vi "Dresden R2R Sputter 03.02.2018 IY24.vi"() -> ()   [LabVIEW 2009] (continued)
              }
            }
          }
          frame #3 {
            # "ROUTINE CHECK"
            n22291 = local read "Semi"() -> (w23224:bool)
            n22292 = case shown="False" w23224 {
              frame #0 {
                n22293 = stacked-sequence {
                  frame #0 {
                    n22294 = local read "Semi"() -> (w23225:bool)
                    n22295 = case shown="False" w23225 {
                      frame #0 {
                        w23226 = TRUE ("Visible")
                        n22296 = local write "system_status"("Start up was completed." ("system_status")) -> ()
                        n22297 = property on="final_mes_tab" class="TabCtl (strict)"("Visible"=w23226) -> ()  [unwired: 2 in, 2 out]
                        n22298 = local write "Cnt_Do_Buzzer"(w23226) -> ()
                        n22299 = Wait (ms)(milliseconds to wait=u32 3000 ("millisecond multiple")) -> ()  [unwired: 1 out]
                      }
                      frame #1 {
                      }
                    }
                  }
                  frame #1 {
                    n22300 = local read "Semi"() -> (w23229:bool)
                    n22301 = case shown="False" w23229 {
                      frame #0 {
                        w23230 = FALSE ("Visible")
                        n22302 = local write "system_status"("" ("system_status")) -> ()
                        n22303 = Wait (ms)(milliseconds to wait=u32 3000 ("millisecond multiple")) -> ()  [unwired: 1 out]
                        n22304 = local write "Start_up_ch4"(w23230) -> ()
                        n22305 = local write "Cnt_Do_Buzzer"(w23230) -> ()
                        n22306 = property on="final_mes_tab" class="TabCtl (strict)"("Visible"=w23230) -> ()  [unwired: 2 in, 2 out]
                      }
                      frame #1 {
                      }
                    }
                  }
                  frame #2 {
                    n22307 = local read "Semi"() -> (w23233:bool)
                    n22308 = case shown="False" w23233 {
                      frame #0 {
                        n22309 = stacked-sequence {
                          frame #0 {
                            n22310 = local write "Pps_code_entry"("PF331=" ("system_status")) -> ()
                          }
                          frame #1 {
                            n22311 = Wait (ms)(milliseconds to wait=u32 500) -> ()  [unwired: 1 out]
                          }
                          frame #2 {
                            n22312 = local write "Ppsok"(TRUE ("Ppsok")) -> ()
                          }
                          frame #3 {
                            n22313 = Wait (ms)(milliseconds to wait=u32 1000) -> ()  [unwired: 1 out]
                          }
                        }
                      }
                      frame #1 {
                      }
                    }
                  }
                  frame #3 {
                    n22314 = local read "Semi"() -> (w23238:bool)
                    n22315 = case shown="False" w23238 {
                      frame #0 {
                        n22316 = stacked-sequence {
                          frame #0 {
                            n22317 = local write "Pps_code_entry"("PF227=" ("system_status")) -> ()
                          }
                          frame #1 {
                            n22318 = Wait (ms)(milliseconds to wait=u32 500) -> ()  [unwired: 1 out]
                          }
                          frame #2 {
                            n22319 = local write "Ppsok"(TRUE ("Ppsok")) -> ()
                          }
                          frame #3 {
                            n22320 = Wait (ms)(milliseconds to wait=u32 1000) -> ()  [unwired: 1 out]
                          }
                        }
                      }
                      frame #1 {
                      }
                    }
                  }
                  frame #4 {
                    n22321 = local read "Semi"() -> (w23243:bool)
                    n22322 = case shown="False" w23243 {
                      frame #0 {
                        n22323 = stacked-sequence {
                          frame #0 {
                            n22324 = local write "Pps_code_entry"("PF330=" ("system_status")) -> ()
                          }
                          frame #1 {
                            n22325 = Wait (ms)(milliseconds to wait=u32 500) -> ()  [unwired: 1 out]
                          }
                          frame #2 {
                            n22326 = local write "Ppsok"(TRUE ("Ppsok")) -> ()
                          }
                          frame #3 {
                            n22327 = Wait (ms)(milliseconds to wait=u32 1000) -> ()  [unwired: 1 out]
                          }
                        }
                      }
                      frame #1 {
                      }
                    }
                  }
                  frame #5 {
                    n22328 = local read "Semi"() -> (w23248:bool)
                    n22329 = case shown="False" w23248 {
                      frame #0 {
                        w23249 = TRUE ("P018")
                        n22330 = local write "Ch4_PA35"(w23249) -> ()
                        n22331 = local write "Ch4_PV22"(w23249) -> ()
                        n22332 = Wait (ms)(milliseconds to wait=u32 1000) -> ()  [unwired: 1 out]
                      }
                      frame #1 {
                      }
                    }
                  }
                }
              }
              frame #1 {
              }
            }
          }
        }
      }
    }
    n22333 = case shown="True" "Shutdown_ch4" {
      frame #0 {
      }
      frame #1 {
        n22334 = local read "Semi"() -> (w21677:bool)
        n22335 = case shown="False" w21677 {
          frame #0 {
            n22336 = stacked-sequence {
              frame #0 {
                n22337 = local read "Semi"() -> (w21678:bool)
                n22338 = case shown="False" w21678 {
                  frame #0 {
                    n22339 = stacked-sequence {
                      frame #0 {
                        w21681 = FALSE
                        n22340 = local write "final_process_messages"("Shut Down process was completed." ("final_process_messages")) -> ()
                        n22341 = local write "system_status"("Shutting Down the System" ("system_status")) -> ()
                        n22342 = local write "Clean_shutdown_ch4"(TRUE) -> ()
                        n22343 = Wait (ms)(milliseconds to wait=u32 1000) -> ()  [unwired: 1 out]
                        "Yes 4" <- w21681
                        "No 4" <- w21681
                        "Cancel 4" <- w21681
                        "Close 4" <- w21681
                      }
                      frame #1 {
                        n22344 = call <vilib>:"Three Button Dialog.vi"("Right Button Text (\"Cancel\")"="Cancel" ("Right Button Text (\"Cancel\")"), "Center Button Text (\"No\")"="No" ("Center Button Text (\"No\")"), "Left Button Text (\"Yes\")"="Yes" ("Left Button Text (\"Yes\")"), "message"=" VENT the CHAMBER  \nLOAD or UNLOAD the substrate ? ") -> ("Which Button?"=w21687:T40)  [unwired: 7 in]
                        n22345 = case shown="\"Window Close\"" w21687 {
                          frame #0 {
                            n22346 = local write "Yes 4"(TRUE ("Close")) -> ()
                          }
                          frame #1 {
                            n22347 = local write "Close 4"(TRUE ("Close")) -> ()
                          }
                          frame #2 {
                            n22348 = local write "Cancel 4"(TRUE ("No")) -> ()
                          }
                          frame #3 {
                            n22349 = local write "No 4"(TRUE ("No")) -> ()
                          }
                        }
                      }
                      frame #2 {
                        n22350 = local read "Semi"() -> (w21693:bool)
                        n22351 = case shown="False" w21693 {
                          frame #0 {
                            n22352 = stacked-sequence {
                              frame #0 {
                                n22353 = local write "Error Message"("" ("Error Message")) -> ()
                              }
                              frame #1 {
                                n22354 = Wait (ms)(milliseconds to wait=u32 500) -> ()  [unwired: 1 out]
                              }
                              frame #2 {
                                n22355 = local write "Ppsok"(TRUE ("Ppsok")) -> ()
                              }
                              frame #3 {
                                n22356 = Wait (ms)(milliseconds to wait=u32 500) -> ()  [unwired: 1 out]
                              }
                            }
                          }
                          frame #1 {
                          }
                        }
                      }
                    }
                  }
                  frame #1 {
                  }
                }
              }
              frame #1 {
                n22357 = local read "Semi"() -> (w21698:bool)
                n22358 = case shown="False" w21698 {
                  frame #0 {
                    n22359 = local read "Cancel 4"() -> (w21700:bool)
                    n22360 = local read "Close 4"() -> (w21701:bool)
                    n22361 = Not Or(1:w21700, 2:w21701) -> (0:w21699:bool)
                    n22362 = case shown="True" w21699 {
                      frame #0 {
                        n22363 = local read "Semi"() -> (w21702:bool)
                        n22364 = case shown="False" w21702 {
                          frame #0 {
                          }
                          frame #1 {
                            n22365 = local write "Shutdown_ch4"(FALSE ("Shutdown_ch1")) -> ()
                            n22366 = local write "system_status"("Semi-automatic is active" ("system_status")) -> ()
                          }
                        }
                      }
                      frame #1 {
                        n22367 = local read "Yes 4"() -> (w21707:bool)
                        n22368 = local read "No 4"() -> (w21706:bool)
                        n22369 = Or(x=w21707, y=w21706) -> (x .or. y?=w21705:bool)
                        n22370 = case shown="True" w21705 {
                          frame #0 {
                          }
                          frame #1 {
                            n22371 = stacked-sequence {
                              frame #0 {
                                # "CLOSE & ZERO ROUTINES"
                                n22372 = local read "Semi"() -> (w21708:bool)
                                n22373 = case shown="False" w21708 {
                                frame #0 {
                                n22374 = stacked-sequence {
                                frame #0 {
                                n22375 = local read "Semi"() -> (w21709:bool)
                                n22376 = case shown="False" w21709 {
                                frame #0 {
                                w21711 = TRUE ("Dc_auto_off")
                                n22377 = local write "Dc_auto_off"(w21711) -> ()
                                n22378 = local write "Ar_auto_set_zero_ch4"(w21711) -> ()
                                n22379 = local write "system_status"("Shut Down in Progress for Chamber 4" ("system_status")) -> ()
                                n22380 = local write "final_process_messages"("Shut Down Process was completed for  Chamber 4." ("final_process_messages")) -> ()
                                n22381 = local write "Ch4_Sov_Ar_do"(FALSE ("Dc_auto_off")) -> ()
                                }
                                frame #1 {
                                }
                                }
                                }
                                frame #1 {
                                n22382 = local read "Semi"() -> (w21714:bool)
                                n22383 = case shown="False" w21714 {
                                frame #0 {
                                n22384 = Wait (ms)(milliseconds to wait=u32 2500) -> ()  [unwired: 1 out]
                                }
                                frame #1 {
                                }
                                }
                                }
                                frame #2 {
                                n22385 = local read "Semi"() -> (w21716:bool)
                                n22386 = case shown="False" w21716 {
                                frame #0 {
                                n22387 = local write "Ch4_Sov_Ar_do"(FALSE ("Ch1_Sov_Ar_do")) -> ()
                                n22388 = Wait (ms)(milliseconds to wait=u32 2500) -> ()  [unwired: 1 out]
                                n22389 = local write "RF_auto_off"(TRUE ("RF_auto_off")) -> ()
                                }
                                frame #1 {
                                }
                                }
                                }
                                frame #3 {
                                n22390 = local read "Semi"() -> (w21720:bool)
                                n22391 = case shown="False" w21720 {
                                frame #0 {
                                n22392 = Wait (ms)(milliseconds to wait=u32 1000) -> ()  [unwired: 1 out]
                                }
                                frame #1 {
                                }
                                }
                                }
                                }
                                }
                                frame #1 {
                                }
                                }
                              }
                              frame #1 {
                                # "STOP TP"
                                n22393 = local read "Semi"() -> (w21722:bool)
                                n22394 = case shown="False" w21722 {
                                frame #0 {
                                n22395 = stacked-sequence {
                                frame #0 {
                                n22396 = local read "Semi"() -> (w21723:bool)
                                n22397 = case shown="False" w21723 {
                                frame #0 {
                                n22398 = stacked-sequence {
                                frame #0 {
                                n22399 = local read "Semi"() -> (w21724:bool)
                                n22400 = case shown="False" w21724 {
                                frame #0 {
                                n22401 = local write "Tp4_auto_stop"(TRUE ("Tp1_auto_start")) -> ()
                                }
                                frame #1 {
                                }
                                }
                                }
                                frame #1 {
                                n22402 = local read "Semi"() -> (w21726:bool)
                                n22403 = case shown="False" w21726 {
                                frame #0 {
                                n22404 = Wait (ms)(milliseconds to wait=u32 1000) -> ()  [unwired: 1 out]
                                }
                                frame #1 {
                                }
                                }
                                }
                                frame #2 {
                                n22405 = local read "Semi"() -> (w21728:bool)
                                n22406 = case shown="False" w21728 {
                                frame #0 {
                                n22407 = while {
                                i -> [w21734]
                                stop <- w21730 stop-if-true
                                n22408 = local read "Tp4_stopped"() -> (w21732:bool)
                                n22409 = Greater?(x=w21734, y=120) -> (0:w21733:bool)
                                n22410 = local read "Semi"() -> (w21731:bool)
                                n22411 = Compound Arithmetic op=OR(w21731, w21732, w21733) -> (w21730:bool)
                                n22412 = Wait (ms)(milliseconds to wait=u32 500) -> ()  [unwired: 1 out]
                                }
                                }
                                frame #1 {
                                }
                                }
                                }
                                frame #3 {
                                n22413 = local read "Semi"() -> (w21736:bool)
                                n22414 = case shown="False" w21736 {
                                frame #0 {
                                n22415 = local read "Tp4_stopped"() -> (w21737:bool)
                                n22416 = case shown="False" w21737 {
                                frame #0 {
                                n22417 = local write "Tp4_auto_stop"(TRUE ("Pc_bv1_auto_open")) -> ()
                                }
                                frame #1 {
                                }
                                }
                                }
                                frame #1 {
                                }
                                }
                                }
                                frame #4 {
                                n22418 = local read "Semi"() -> (w21739:bool)
                                n22419 = case shown="False" w21739 {
                                frame #0 {
                                n22420 = local read "Tp4_stopped"() -> (w21740:bool)
                                n22421 = case shown="False" w21740 {
                                frame #0 {
                                n22422 = Wait (ms)(milliseconds to wait=u32 1000) -> ()  [unwired: 1 out]
                                }
                                frame #1 {
                                }
                                }
                                }
                                frame #1 {
                                }
                                }
                                }
                                frame #5 {
                                n22423 = local read "Semi"() -> (w21742:bool)
                                n22424 = case shown="False" w21742 {
                                frame #0 {
                                n22425 = while {
                                i -> [w21748]
                                stop <- w21744 stop-if-true
                                n22426 = local read "Tp4_stopped"() -> (w21746:bool)
                                n22427 = Greater?(x=w21748, y=120) -> (0:w21747:bool)
                                n22428 = local read "Semi"() -> (w21745:bool)
                                n22429 = Compound Arithmetic op=OR(w21745, w21746, w21747) -> (w21744:bool)
                                n22430 = Wait (ms)(milliseconds to wait=u32 500) -> ()  [unwired: 1 out]
                                }
                                }
                                frame #1 {
                                }
                                }
                                }
                                frame #6 {
                                n22431 = local read "Semi"() -> (w21750:bool)
                                n22432 = case shown="False" w21750 {
                                frame #0 {
                                n22433 = local read "Tp4_stopped"() -> (w21751:bool)
                                n22434 = case shown="False" w21751 {
                                frame #0 {
                                n22435 = local write "Error Message"("Shut Down process  cancelled\nbecause  TP not stopped.\nPlease check TP4  connections." ("Error Message")) -> ()
                                n22436 = local write "Semi"(TRUE ("Semi")) -> ()
                                }
                                frame #1 {
                                }
                                }
                                }
                                frame #1 {
                                }
                                }
                                }
                                }
                                }
                                frame #1 {
                                }
                                }
                                }
                                frame #1 {
                                n22437 = local read "Semi"() -> (w21754:bool)
                                n22438 = case shown="False" w21754 {
                                frame #0 {
                                n22439 = local write "Ch4_Sd1"(TRUE ("Ch1_Sd0")) -> ()
                                n22440 = Wait (ms)(milliseconds to wait=u32 1000) -> ()  [unwired: 1 out]
                                }
                                frame #1 {
                                }
                                }
                                }
                                }
                                }
                                frame #1 {
                                }
                                }
                              }
                              frame #2 {
                                # "CLOSE CC"
                                n22441 = local read "Semi"() -> (w21757:bool)
                                n22442 = case shown="False" w21757 {
                                frame #0 {
                                n22443 = stacked-sequence {
                                frame #0 {
                                n22444 = local read "Semi"() -> (w21758:bool)
                                n22445 = case shown="False" w21758 {
                                frame #0 {
                                n22446 = while {
                                i -> [w21764]
                                stop <- w21759 stop-if-true
                                n22447 = Greater?(x=w21764, y=25) -> (0:w21763:bool)
                                n22448 = case shown="True" w21763 {
                                frame #0 {
                                }
                                frame #1 {
                                n22449 = local write "Error Message"("Shut Down Process  cancelled\nbecause  CC not closed.\nPlease check CH4-CC connections." ("Error Message")) -> ()
                                n22450 = local write "Semi"(TRUE ("Semi")) -> ()
                                }
                                }
                                n22451 = local read "Ch4_Cc_on_off_di"() -> (w21762:bool)
                                n22452 = case shown="True" w21762 {
                                tunnel: [TRUE FALSE] -> w21760
                                frame #0 {
                                }
                                frame #1 {
                                n22453 = local write "Ch4_Cc_on_off_do"(FALSE ("Ch1_Ch_cc_on_off_di")) -> ()
                                n22454 = Wait Until Next ms Multiple(millisecond multiple=u32 200) -> ()  [unwired: 1 out]
                                }
                                }
                                n22455 = local read "Semi"() -> (w21761:bool)
                                n22456 = Or(x=w21760, y=w21761) -> (x .or. y?=w21759:bool)
                                }
                                }
                                frame #1 {
                                }
                                }
                                }
                                frame #1 {
                                n22457 = local read "Semi"() -> (w21772:bool)
                                n22458 = case shown="False" w21772 {
                                frame #0 {
                                n22459 = local write "Ch4_Sd2"(TRUE ("Ch1_Sd1")) -> ()
                                n22460 = Wait (ms)(milliseconds to wait=u32 1000) -> ()  [unwired: 1 out]
                                }
                                frame #1 {
                                }
                                }
                                }
                                }
                                }
                                frame #1 {
                                }
                                }
                              }
                              frame #3 {
                                # "CLOSE BG-BV"
                                n22461 = local read "Semi"() -> (w21775:bool)
                                n22462 = case shown="False" w21775 {
                                frame #0 {
                                n22463 = stacked-sequence {
                                frame #0 {
                                n22464 = local read "Semi"() -> (w21776:bool)
                                n22465 = case shown="False" w21776 {
                                frame #0 {
                                n22466 = while {
                                i -> [w21782]
                                stop <- w21777 stop-if-true
                                n22467 = Greater?(x=w21782, y=25) -> (0:w21781:bool)
                                n22468 = case shown="True" w21781 {
                                frame #0 {
                                }
                                frame #1 {
                                n22469 = local write "Error Message"("Shut Down Process  cancelled\nbecause  BG-BV not closed.\nPlease check BG-BV4  connections." ("Error Message")) -> ()
                                n22470 = local write "Semi"(TRUE ("Semi")) -> ()
                                }
                                }
                                n22471 = local read "Ch4_Bg_bv_di"() -> (w21780:bool)
                                n22472 = case shown="True" w21780 {
                                tunnel: [TRUE FALSE] -> w21778
                                frame #0 {
                                }
                                frame #1 {
                                n22473 = Wait Until Next ms Multiple(millisecond multiple=u32 200) -> ()  [unwired: 1 out]
                                n22474 = local write "Ch4_Bg_bv_do"(FALSE ("Ch1_Ch_cc_on_off_di")) -> ()
                                }
                                }
                                n22475 = local read "Semi"() -> (w21779:bool)
                                n22476 = Or(x=w21778, y=w21779) -> (x .or. y?=w21777:bool)
                                }
                                }
                                frame #1 {
                                }
                                }
                                }
                                frame #1 {
                                n22477 = local read "Semi"() -> (w21790:bool)
                                n22478 = case shown="False" w21790 {
                                frame #0 {
                                n22479 = Wait (ms)(milliseconds to wait=u32 1000) -> ()  [unwired: 1 out]
                                n22480 = local write "Ch4_Sd3"(TRUE ("Ch1_Sd1 2")) -> ()
                                }
                                frame #1 {
                                }
                                }
                                }
                                }
                                }
                                frame #1 {
                                }
                                }
                              }
                              frame #4 {
                                n22481 = local read "Yes 4"() -> (w21793:bool)
                                n22482 = case shown="True" w21793 {
                                frame #0 {
                                # "CLOSE PC-BV"
                                n22483 = local read "Semi"() -> (w21794:bool)
                                n22484 = case shown="False" w21794 {
                                frame #0 {
                                n22485 = stacked-sequence {
                                frame #0 {
                                n22486 = local read "Semi"() -> (w21795:bool)
                                n22487 = case shown="False" w21795 {
                                frame #0 {
                                n22488 = stacked-sequence {
                                frame #0 {
                                n22489 = local read "Semi"() -> (w21796:bool)
                                n22490 = case shown="False" w21796 {
                                frame #0 {
                                n22491 = local write "Pc_bv4_auto_close"(TRUE ("Tp1_auto_start")) -> ()
                                }
                                frame #1 {
                                }
                                }
                                }
                                frame #1 {
                                n22492 = local read "Semi"() -> (w21798:bool)
                                n22493 = case shown="False" w21798 {
                                frame #0 {
                                n22494 = Wait (ms)(milliseconds to wait=u32 1000) -> ()  [unwired: 1 out]
                                }
                                frame #1 {
                                }
                                }
                                }
                                frame #2 {
                                n22495 = local read "Semi"() -> (w21800:bool)
                                n22496 = case shown="False" w21800 {
                                frame #0 {
                                n22497 = while {
                                i -> [w21806]
                                stop <- w21802 stop-if-true
                                n22498 = local read "Pc_bv_closed_ch4"() -> (w21804:bool)
                                n22499 = Greater?(x=w21806, y=120) -> (0:w21805:bool)
                                n22500 = local read "Semi"() -> (w21803:bool)
                                n22501 = Compound Arithmetic op=OR(w21803, w21804, w21805) -> (w21802:bool)
                                n22502 = Wait (ms)(milliseconds to wait=u32 500) -> ()  [unwired: 1 out]
                                }
                                }
                                frame #1 {
                                }
                                }
                                }
                                frame #3 {
                                n22503 = local read "Semi"() -> (w21808:bool)
                                n22504 = case shown="False" w21808 {
                                frame #0 {
                                n22505 = local read "Pc_bv_closed_ch4"() -> (w21809:bool)
                                n22506 = case shown="False" w21809 {
                                frame #0 {
                                n22507 = local write "Pc_bv4_auto_close"(TRUE ("Pc_bv1_auto_open")) -> ()
                                }
                                frame #1 {
                                }
                                }
                                }
                                frame #1 {
                                }
                                }
                                }
                                frame #4 {
                                n22508 = local read "Semi"() -> (w21811:bool)
                                n22509 = case shown="False" w21811 {
                                frame #0 {
                                n22510 = local read "Pc_bv_closed_ch4"() -> (w21812:bool)
                                n22511 = case shown="False" w21812 {
                                frame #0 {
                                n22512 = Wait (ms)(milliseconds to wait=u32 1000) -> ()  [unwired: 1 out]
                                }
                                frame #1 {
                                }
                                }
                                }
                                frame #1 {
                                }
                                }
                                }
                                frame #5 {
                                n22513 = local read "Semi"() -> (w21814:bool)
                                n22514 = case shown="False" w21814 {
                                frame #0 {
                                n22515 = while {
                                i -> [w21820]
                                stop <- w21816 stop-if-true
                                n22516 = local read "Pc_bv_closed_ch4"() -> (w21818:bool)
                                n22517 = Greater?(x=w21820, y=120) -> (0:w21819:bool)
                                n22518 = local read "Semi"() -> (w21817:bool)
                                n22519 = Compound Arithmetic op=OR(w21817, w21818, w21819) -> (w21816:bool)
                                n22520 = Wait (ms)(milliseconds to wait=u32 500) -> ()  [unwired: 1 out]
                                }
                                }
                                frame #1 {
                                }
                                }
                                }
                                frame #6 {
                                n22521 = local read "Semi"() -> (w21822:bool)
                                n22522 = case shown="False" w21822 {
                                frame #0 {
                                n22523 = local read "Pc_bv_closed_ch4"() -> (w21823:bool)
                                n22524 = case shown="False" w21823 {
                                frame #0 {
                                n22525 = local write "Error Message"("Shut Down process  cancelled\nbecause  PC-BV not opened.\nPlease check PC-BV4  connections." ("Error Message")) -> ()
                                n22526 = local write "Semi"(TRUE ("Semi")) -> ()
                                }
                                frame #1 {
                                }
                                }
                                }
                                frame #1 {
                                }
                                }
                                }
                                }
                                }
                                frame #1 {
                                }
                                }
                                }
                                frame #1 {
                                n22527 = local read "Semi"() -> (w21826:bool)
                                n22528 = case shown="False" w21826 {
                                frame #0 {
                                n22529 = Wait (ms)(milliseconds to wait=u32 1000) -> ()  [unwired: 1 out]
                                n22530 = local write "Ch4_Sd4"(TRUE ("Ch1_Sd2")) -> ()
                                }
                                frame #1 {
                                }
                                }
                                }
                                }
                                }
                                frame #1 {
                                }
                                }
                                }
                                frame #1 {
                                # "OPEN PC-BV"
                                n22531 = local read "Semi"() -> (w21829:bool)
                                n22532 = case shown="False" w21829 {
                                frame #0 {
                                n22533 = stacked-sequence {
                                frame #0 {
                                n22534 = local read "Semi"() -> (w21830:bool)
                                n22535 = case shown="False" w21830 {
                                frame #0 {
                                n22536 = stacked-sequence {
                                frame #0 {
                                n22537 = local read "Semi"() -> (w21831:bool)
                                n22538 = case shown="False" w21831 {
                                frame #0 {
                                n22539 = local write "Pc_bv4_auto_open"(TRUE ("Tp1_auto_start")) -> ()
                                }
                                frame #1 {
                                }
                                }
                                }
                                frame #1 {
                                n22540 = local read "Semi"() -> (w21833:bool)
                                n22541 = case shown="False" w21833 {
                                frame #0 {
                                n22542 = Wait (ms)(milliseconds to wait=u32 1000) -> ()  [unwired: 1 out]
                                }
                                frame #1 {
                                }
                                }
                                }
                                frame #2 {
                                n22543 = local read "Semi"() -> (w21835:bool)
                                n22544 = case shown="False" w21835 {
                                frame #0 {
                                n22545 = while {
                                i -> [w21841]
                                stop <- w21837 stop-if-true
                                n22546 = local read "Pc_bv_opened_ch4"() -> (w21839:bool)
                                n22547 = Greater?(x=w21841, y=120) -> (0:w21840:bool)
                                n22548 = local read "Semi"() -> (w21838:bool)
                                n22549 = Compound Arithmetic op=OR(w21838, w21839, w21840) -> (w21837:bool)
                                n22550 = Wait (ms)(milliseconds to wait=u32 500) -> ()  [unwired: 1 out]
                                }
                                }
                                frame #1 {
                                }
                                }
                                }
                                frame #3 {
                                n22551 = local read "Semi"() -> (w21843:bool)
                                n22552 = case shown="False" w21843 {
                                frame #0 {
                                n22553 = local read "Pc_bv_opened_ch4"() -> (w21844:bool)
                                n22554 = case shown="False" w21844 {
                                frame #0 {
                                n22555 = local write "Pc_bv4_auto_close"(TRUE ("Pc_bv1_auto_open")) -> ()
                                }
                                frame #1 {
                                }
                                }
                                }
                                frame #1 {
                                }
                                }
                                }
                                frame #4 {
                                n22556 = local read "Semi"() -> (w21846:bool)
                                n22557 = case shown="False" w21846 {
                                frame #0 {
                                n22558 = local read "Pc_bv_opened_ch4"() -> (w21847:bool)
                                n22559 = case shown="False" w21847 {
                                frame #0 {
                                n22560 = Wait (ms)(milliseconds to wait=u32 1000) -> ()  [unwired: 1 out]
                                }
                                frame #1 {
                                }
                                }
                                }
                                frame #1 {
                                }
                                }
                                }
                                frame #5 {
                                n22561 = local read "Semi"() -> (w21849:bool)
                                n22562 = case shown="False" w21849 {
                                frame #0 {
                                n22563 = while {
                                i -> [w21855]
                                stop <- w21851 stop-if-true
                                n22564 = local read "Pc_bv_opened_ch4"() -> (w21853:bool)
                                n22565 = Greater?(x=w21855, y=120) -> (0:w21854:bool)
                                n22566 = local read "Semi"() -> (w21852:bool)
                                n22567 = Compound Arithmetic op=OR(w21852, w21853, w21854) -> (w21851:bool)
                                n22568 = Wait (ms)(milliseconds to wait=u32 500) -> ()  [unwired: 1 out]
                                }
                                }
                                frame #1 {
                                }
                                }
                                }
                                frame #6 {
                                n22569 = local read "Semi"() -> (w21857:bool)
                                n22570 = case shown="False" w21857 {
                                frame #0 {
                                n22571 = local read "Pc_bv_opened_ch4"() -> (w21858:bool)
                                n22572 = case shown="False" w21858 {
                                frame #0 {
                                n22573 = local write "Error Message"("Shut Down process  cancelled\nbecause  PC-BV not opened.\nPlease check PC-BV4 connections." ("Error Message")) -> ()
                                n22574 = Wait (ms)(milliseconds to wait=u32 1000) -> ()  [unwired: 1 out]
                                }
                                frame #1 {
                                }
                                }
                                }
                                frame #1 {
                                }
                                }
                                }
                                }
                                }
                                frame #1 {
                                }
                                }
                                }
                                frame #1 {
                                n22575 = local read "Semi"() -> (w21861:bool)
                                n22576 = case shown="False" w21861 {
                                frame #0 {
                                n22577 = Wait (ms)(milliseconds to wait=u32 1000) -> ()  [unwired: 1 out]
                                n22578 = local write "Ch4_Sd5"(TRUE ("Ch1_Sd2")) -> ()
                                }
                                frame #1 {
                                }
                                }
                                }
                                }
                                }
                                frame #1 {
                                }
                                }
                                }
                                }
                              }
                              frame #5 {
                                # "CLOSE TP-BV"
                                n22579 = local read "Semi"() -> (w21864:bool)
                                n22580 = case shown="False" w21864 {
                                frame #0 {
                                n22581 = stacked-sequence {
                                frame #0 {
                                n22582 = local read "Semi"() -> (w21865:bool)
                                n22583 = case shown="False" w21865 {
                                frame #0 {
                                n22584 = while {
                                i -> [w21871]
                                stop <- w21866 stop-if-true
                                n22585 = Greater?(x=w21871, y=25) -> (0:w21870:bool)
                                n22586 = case shown="True" w21870 {
                                frame #0 {
                                }
                                frame #1 {
                                n22587 = local write "Error Message"("Shut Down Process  cancelled\nbecause  TP-BV not closed.\nPlease check TP-BV4 connections." ("Error Message")) -> ()
                                n22588 = local write "Semi"(TRUE ("Semi")) -> ()
                                }
                                }
                                n22589 = local read "Ch4_Tp_bv_di"() -> (w21869:bool)
                                n22590 = case shown="True" w21869 {
                                tunnel: [TRUE FALSE] -> w21867
                                frame #0 {
                                }
                                frame #1 {